vi "Dresden R2R Sputter 03.02.2018 IY24.vi"() -> ()   [LabVIEW 2009] (continued)
            n9500 = local read "Ch1_Tp_bv_do"() -> (w15535:bool)
            n9501 = local read "Ch1_Tp_bv_di"() -> (w15536:bool)
            n9502 = Exclusive Or(1:w15535, 2:w15536) -> (0:w15552:bool)
            n9503 = feedback #324() -> (w15551:bool)  [unwired: 1 in]
            n9504 = case shown="True" w15552 {
              tunnel: [TRUE FALSE] -> w15550
              tunnel: w15551 -> [_ w15589]
              tunnel: [FALSE w15586] -> w15534
              frame #0 {
              }
              frame #1 {
                n9505 = call "Elapsed Time96"("Reset"=w15589) -> ("Elapsed Time (s)"=w15588:dbl)  [unwired: 11 in, 7 out]
                n9506 = Greater?(x=w15588, y=5.0) -> (0:w15586:bool)
              }
            }
            n9507 = local write "Ch1_Tp_bv_fail"(w15534) -> ()
            n9508 = local read "Ch1_Bg_bv_di"() -> (w15533:bool)
            n9509 = local read "Ch1_Bg_bv_do"() -> (w15532:bool)
            n9510 = Exclusive Or(1:w15532, 2:w15533) -> (0:w15547:bool)
            n9511 = feedback #325() -> (w15548:bool)  [unwired: 1 in]
            n9512 = case shown="True" w15547 {
              tunnel: [TRUE FALSE] -> w15549
              tunnel: w15548 -> [_ w15582]
              tunnel: [FALSE w15579] -> w15522
              frame #0 {
              }
              frame #1 {
                n9513 = call "Elapsed Time97"("Reset"=w15582) -> ("Elapsed Time (s)"=w15581:dbl)  [unwired: 11 in, 7 out]
                n9514 = Greater?(x=w15581, y=5.0) -> (0:w15579:bool)
              }
            }
            n9515 = local write "ch1_bg_bv_fail_top"(w15522) -> ()
            n9516 = local write "Ch1_Bg_bv_fail"(w15522) -> ()
            n9517 = local read "Ch1_Ch_vbv_do"() -> (w15530:bool)
            n9518 = local read "Ch1_Ch_vbv_di"() -> (w15531:bool)
            n9519 = Exclusive Or(1:w15530, 2:w15531) -> (0:w15546:bool)
            n9520 = feedback #326() -> (w15545:bool)  [unwired: 1 in]
            n9521 = case shown="True" w15546 {
              tunnel: [TRUE FALSE] -> w15544
              tunnel: w15545 -> [_ w15575]
              tunnel: [FALSE w15572] -> w15529
              frame #0 {
              }
              frame #1 {
                n9522 = call "Elapsed Time98"("Reset"=w15575) -> ("Elapsed Time (s)"=w15574:dbl)  [unwired: 11 in, 7 out]
                n9523 = Greater?(x=w15574, y=5.0) -> (0:w15572:bool)
              }
            }
            n9524 = local write "Ch1_Ch_vbv_fail"(w15529) -> ()
            n9525 = local read "Ch1_Pl_vbv_do"() -> (w15526:bool)
            n9526 = local read "Ch1_Pl_vbv_di"() -> (w15527:bool)
            n9527 = Exclusive Or(1:w15526, 2:w15527) -> (0:w15523:bool)
            n9528 = feedback #327() -> (w15543:bool)  [unwired: 1 in]
            n9529 = case shown="True" w15523 {
              tunnel: [TRUE FALSE] -> w15542
              tunnel: w15543 -> [_ w15568]
              tunnel: [FALSE w15565] -> w15528
              frame #0 {
              }
              frame #1 {
                n9530 = call "Elapsed Time100"("Reset"=w15568) -> ("Elapsed Time (s)"=w15567:dbl)  [unwired: 11 in, 7 out]
                n9531 = Greater?(x=w15567, y=5.0) -> (0:w15565:bool)
              }
            }
            n9532 = local write "Ch1_Pl_vbv_fail"(w15528) -> ()
            n9533 = local read "Ch1_Cc_on_off_di"() -> (w15525:bool)
            n9534 = local read "Ch1_Cc_on_off_do"() -> (w15524:bool)
            n9535 = feedback #328() -> (w15540:bool)  [unwired: 1 in]
            n9536 = Exclusive Or(1:w15524, 2:w15525) -> (0:w15541:bool)
            n9537 = case shown="True" w15541 {
              tunnel: [TRUE FALSE] -> w15539
              tunnel: w15540 -> [_ w15561]
              tunnel: [FALSE w15558] -> w15521
              frame #0 {
              }
              frame #1 {
                n9538 = call "Elapsed Time102"("Reset"=w15561) -> ("Elapsed Time (s)"=w15560:dbl)  [unwired: 11 in, 7 out]
                n9539 = Greater?(x=w15560, y=5.0) -> (0:w15558:bool)
              }
            }
            n9540 = local write "ch1_cc_fail_top"(w15521) -> ()
            n9541 = local write "Ch1_Ch_cc_fail"(w15521) -> ()
          }
        }
        n9542 = case shown="False" w15450 {
          frame #0 {
            n9543 = local read "Ch1_Sov_Ar_do"() -> (w15492:bool)
            n9544 = local read "Ch1_Sov_Ar_di"() -> (w15493:bool)
            n9545 = Exclusive Or(1:w15492, 2:w15493) -> (0:w15494:bool)
            n9546 = feedback #329() -> (w15495:bool)  [unwired: 1 in]
            n9547 = case shown="True" w15494 {
              tunnel: [TRUE FALSE] -> w15496
              tunnel: w15495 -> [_ w15516]
              tunnel: [FALSE w15513] -> w15479
              frame #0 {
              }
              frame #1 {
                n9548 = call "Elapsed Time103"("Reset"=w15516) -> ("Elapsed Time (s)"=w15515:dbl)  [unwired: 11 in, 7 out]
                n9549 = Greater?(x=w15515, y=5.0) -> (0:w15513:bool)
              }
            }
            n9550 = local write "ch1_sov_Ar_fail_top"(w15479) -> ()
            n9551 = local read "Ch1_Trns_gv_open_di"() -> (w15488:bool)
            n9552 = local read "Ch1_Trns_gv_open_do"() -> (w15487:bool)
            n9553 = Exclusive Or(1:w15487, 2:w15488) -> (0:w15491:bool)
            n9554 = feedback #330() -> (w15490:bool)  [unwired: 1 in]
            n9555 = case shown="True" w15491 {
              tunnel: [TRUE FALSE] -> w15489
              tunnel: w15490 -> [_ w15509]
              tunnel: [FALSE w15506] -> w15486
              frame #0 {
              }
              frame #1 {
                n9556 = call "Elapsed Time135"("Reset"=w15509) -> ("Elapsed Time (s)"=w15508:dbl)  [unwired: 11 in, 7 out]
                n9557 = Greater?(x=w15508, y=60.0) -> (0:w15506:bool)
              }
            }
            n9558 = local write "Trns_gv1_2_fail"(w15486) -> ()
            n9559 = local write "gv top failed_ch2_1"(w15486) -> ()
            n9560 = local write "gv front failed_ch2_1"(w15486) -> ()
            n9561 = local write "gv top failed ch1"(w15486) -> ()
            n9562 = local write "gv front failed ch1_2"(w15486) -> ()
            n9563 = local read "Ch1_Cst_fix_down_di"() -> (w15484:bool)
            n9564 = local read "Ch1_Cst_fix_do"() -> (w15485:bool)
            n9565 = Exclusive Or(1:w15484, 2:w15485) -> (0:w15481:bool)
            n9566 = feedback #331() -> (w15483:bool)  [unwired: 1 in]
            n9567 = case shown="True" w15481 {
              tunnel: [TRUE FALSE] -> w15482
              tunnel: w15483 -> [_ w15502]
              tunnel: [FALSE w15499] -> w15480
              frame #0 {
              }
              frame #1 {
                n9568 = call "Elapsed Time186"("Reset"=w15502) -> ("Elapsed Time (s)"=w15501:dbl)  [unwired: 11 in, 7 out]
                n9569 = Greater?(x=w15501, y=60.0) -> (0:w15499:bool)
              }
            }
            n9570 = local write "chamber 1 top piston failed ch1"(w15480) -> ()
          }
          frame #1 {
            w15518 = TRUE
            n9571 = local write "Trns_gv1_2_fail"(w15518) -> ()
            n9572 = local write "ch1_sov_Ar_fail_top"(w15518) -> ()
            n9573 = local write "gv top failed_ch2_1"(w15518) -> ()
            n9574 = local write "gv front failed_ch2_1"(w15518) -> ()
            n9575 = local write "gv top failed ch1"(w15518) -> ()
            n9576 = local write "gv front failed ch1_2"(w15518) -> ()
            n9577 = local write "chamber 1 top piston failed ch1"(w15518) -> ()
          }
        }
        n9578 = case shown="True" w15448 {
          frame #0 {
            n9579 = disable-structure shown="Disabled" {
              frame #0 {
                n9580 = local read "Ch1_Right_limit_di"() -> (w15454:bool)
                n9581 = local read "Ch1_Do_4_4"() -> (w15455:bool)
                n9582 = Exclusive Or(1:w15455, 2:w15454) -> (0:w15453:bool)
                n9583 = feedback #332() -> (w15452:bool)  [unwired: 1 in]
                n9584 = case shown="True" w15453 {
                  tunnel: [TRUE FALSE] -> w15451
                  tunnel: w15452 -> [_ w15462]
                  tunnel: [FALSE w15459] -> w15456
                  frame #0 {
                  }
                  frame #1 {
                    n9585 = call "Elapsed Time108"("Reset"=w15462) -> ("Elapsed Time (s)"=w15461:dbl)  [unwired: 11 in, 7 out]
                    n9586 = Greater?(x=w15461, y=5.0) -> (0:w15459:bool)
                  }
                }
                n9587 = local write "Ch1_Bp_bv_fail_R"(w15456) -> ()
              }
              frame #1 {
              }
            }
          }
          frame #1 {
            n9588 = disable-structure shown="Disabled" {
              frame #0 {
                n9589 = local write "Ch1_Bp_bv_fail_R"(FALSE ("Bp_bv_fail(ch1)R")) -> ()
              }
              frame #1 {
              }
            }
          }
        }
      }
    }
    n9590 = Wait Until Next ms Multiple(millisecond multiple=u32 200) -> ()  [unwired: 1 out]
  }
  n9591 = while {
    tunnel: w804 -> [w15654]
    tunnel: w803 -> [w15653]
    tunnel: [w15652] -> w802
    tunnel: [w15651] -> w801
    tunnel: w737 -> [w15606]
    tunnel: w736 -> [w15605]
    tunnel: [w15604] -> w735
    tunnel: [w15603] -> w734
    tunnel: w27 -> [w15602]
    tunnel: w26 -> [w15601]
    tunnel: [w15599] -> w25
    tunnel: [w15598] -> w24
    stop <- i16? 0 stop-if-true
    # "According to manual, all starting addresses must be used increment"
    n9592 = Wait Until Next ms Multiple(millisecond multiple=i32? 300) -> ()  [unwired: 1 out]
    n9593 = Or(x="TC1_set", y="TC1_auto_set") -> (x .or. y?=w15636)
    n9594 = Or(x="TC2_set", y="TC2_auto_set") -> (x .or. y?=w15612)
    n9595 = Build Array(i16? 0, w15636, "TC1_open_loop_set", "TC1_close_loop_set", "TC1_P_set", "TC1_I_set", "TC1_D_set", "TC1_speed_gain_set", "TC1_speed_coefficient_set", "TC1_overspeed_set", "TC1_AO1_upper_limit_set", "TC1_AO1_bottom_limit_set", "TC1_AO1_polarity(neg_to_pos)", "TC1_AO1_polarity(pos_to_neg)", "TC1_display_tension_set", "TC1_display_AO1_set", "TC1_display_tension_actual", "TC1_display_AO1_actual", "TC1_tare_function") -> (w15657)
    n9596 = Build Array(i16? 0, w15612, "TC2_open_loop_set", "TC2_close_loop_set", "TC2_P_set", "TC2_I_set", "TC2_D_set", "TC2_speed_gain_set", "TC2_speed_coefficient_set", "TC2_overspeed_set", "TC2_AO1_upper_limit_set", "TC2_AO1_bottom_limit_set", "TC2_AO1_polarity(neg_to_pos)", "TC2_AO1_polarity(pos_to_neg)", "TC2_display_tension_set", "TC2_display_AO1_set", "TC2_display_tension_actual", "TC2_display_AO1_actual", "TC2_tare_function") -> (w15629)
    n9597 = Boolean Array To Number(Boolean array=w15657) -> (number=w15658)
    n9598 = Boolean Array To Number(Boolean array=w15629) -> (number=w15630)
    n9599 = case shown="True" "Counter_reset" {
      tunnel: w15602 -> [w15667 w15676]
      tunnel: w15601 -> [w15666 w15675]
      tunnel: [w15665 w15674] -> w15599
      tunnel: [w15664 w15673] -> w15598
      frame #0 {
        n9600 = call-poly <vilib>:"MB Serial Master Query (poly).vi"(0:w15667, 1:i16? 1000 ("Starting Address"), 2:i16? 13 ("Quantity"), 5:w15666, 6:data[3B] ("Serial Parameters")) -> (14:w15665, 15:w15663, 19:w15664)  [unwired: 1 in, 11 out]
        n9601 = Index Array(array=w15663, index=i32? 3) -> (element=→"Counter_read_data")
      }
      frame #1 {
        n9602 = local write "Counter_reset"(i16? 0 ("Counter_reset")) -> ()
        n9603 = call-poly <vilib>:"MB Serial Master Query (poly).vi"(0:w15676, 1:data[3B] ("Starting Address"), 2:T/1, 5:w15675, 6:data[3B] ("Serial Parameters")) -> (14:w15674, 19:w15673)  [unwired: 1 in, 12 out]
      }
    }
    n9604 = Mantissa & Exponent(0:w15658) -> (2:w15656)  [unwired: 1 out]
    n9605 = Mantissa & Exponent(0:w15630) -> (2:w15628)  [unwired: 1 out]
    n9606 = case shown="1" w15656 {
      tunnel: w15654 -> [w16130 w16153 w16175 w16197 w16219 w16241 w16263 w16285 w16307 w16329 w16351 w16373 w16395 w16417 w16439 w16461 w16483 w16505 w16527]
      tunnel: w15653 -> [w16129 w16152 w16174 w16196 w16218 w16240 w16262 w16284 w16306 w16328 w16350 w16372 w16394 w16416 w16438 w16460 w16482 w16504 w16526]
      tunnel: [w16128 w16156 w16178 w16200 w16222 w16244 w16266 w16288 w16310 w16332 w16354 w16376 w16398 w16420 w16442 w16464 w16486 w16508 w16529] -> w15652
      tunnel: [w16106 w16155 w16177 w16199 w16221 w16243 w16265 w16287 w16309 w16331 w16353 w16375 w16397 w16419 w16441 w16463 w16485 w16507 w16528] -> w15651
      frame #0 {
        n9607 = Increment(x=i16? 296 ("Starting Address")) -> (x+1=w16126)
        n9608 = call <vilib>:"MB Serial Master Query Read Holding Registers (poly).vi"(0:w16130, 1:w16126, 2:i16? 4 ("Quantity"), 5:w16129, 6:data[3B] ("Serial Parameters")) -> (14:w16128, 15:w16107, 19:w16106)  [unwired: 11 in, 1 out]
        n9609 = Index Array(array=w16107, index=data[5B]) -> (element=w16123)
        n9610 = Index Array(array=w16107, index=i32? 2) -> (element=w16121)
        n9611 = Index Array(array=w16107, index=i32? 6) -> (element=w16113)
        n9612 = Type Cast(type=data[5B], x=w16123) -> (*(type *) &x=w16105)
        "TC1_reading_set_value" <- w16105
        n9613 = Type Cast(type=data[5B], x=w16121) -> (*(type *) &x=w16115)
        n9614 = Type Cast(type=data[5B], x=w16113) -> (*(type *) &x=w16109)
        n9615 = Greater?(x=w16115, y=sgl? 0.1) -> (0:w16117)
        n9616 = Divide(x=w16109, y=sgl? 10) -> (x/y=→"TC1_reading_ao_value")
        n9617 = Select(t=w16115, s=w16117, f=data[5B]) -> (s? t:f=→"TC1_measure_value")
        n9618 = stacked-sequence {
          tunnel: w16105 -> [w16132]
          frame #0 {
            n9619 = feedback #333() -> (w16144)  [unwired: 1 in]
            n9620 = feedback #334() -> (w16142)  [unwired: 1 in]
            n9621 = feedback #335() -> (w16141)  [unwired: 1 in]
            n9622 = feedback #336() -> (w16140)  [unwired: 1 in]
            n9623 = feedback #337() -> (w16139)  [unwired: 1 in]
            n9624 = feedback #338() -> (w16138)  [unwired: 1 in]
            n9625 = feedback #339() -> (w16137)  [unwired: 1 in]
            n9626 = feedback #340() -> (w16135)  [unwired: 1 in]
            n9627 = feedback #341() -> (w16136)  [unwired: 1 in]
            n9628 = Compound Arithmetic op=ADD(w16132, w16144, w16142, w16141, w16140, w16139, w16138, w16137, w16135, w16136) -> (w16143)
            n9629 = Divide(x=w16143, y=dbl? 10.0) -> (x/y=→"TC1_Tension_read_set")
          }
        }
      }
      frame #1 {
        w16145 = i16? 0 ("TC1_set")
        w16154 = data[3B] ("Serial Parameters")
        n9630 = Type Cast(type=data[3B], x="TC1_set_value") -> (*(type *) &x=w16146)
        n9631 = Build Array(w16146) -> (w16147)
        n9632 = Increment(x=i16? 142) -> (x+1=w16151)
        n9633 = call <vilib>:"MB Serial Master Query Write Multiple Registers (poly).vi"(0:w16153, 1:w16151, 2:w16147, 5:w16152, 6:w16154) -> (14:w16161, 19:w16160)  [unwired: 12 in, 1 out]
        n9634 = local write "TC1_auto_set"(w16145) -> ()
        n9635 = local write "TC1_set"(w16145) -> ()
        n9636 = Build Array(i32? 49152 ("element")) -> (w16159)
        n9637 = call <vilib>:"MB Serial Master Query Write Multiple Registers (poly).vi"(0:w16161, 1:i16? 320 ("Starting Address"), 2:w16159, 5:w16160, 6:w16154) -> (14:w16165, 19:w16166)  [unwired: 12 in, 1 out]
        n9638 = Build Array(i32? 49407 ("element")) -> (w16162)
        n9639 = call <vilib>:"MB Serial Master Query Write Multiple Registers (poly).vi"(0:w16165, 1:i16? 320 ("Starting Address"), 2:w16162, 5:w16166, 6:w16154) -> (14:w16156, 19:w16155)  [unwired: 12 in, 1 out]
      }
      frame #2 {
        w16176 = data[3B] ("Serial Parameters")
        n9640 = Type Cast(type=data[3B], x="TC1_open_loop_coefficient") -> (*(type *) &x=w16168)
        n9641 = Build Array(w16168) -> (w16169)
        n9642 = Increment(x=i16? 82) -> (x+1=w16173)
        n9643 = call <vilib>:"MB Serial Master Query Write Multiple Registers (poly).vi"(0:w16175, 1:w16173, 2:w16169, 5:w16174, 6:w16176) -> (14:w16183, 19:w16182)  [unwired: 12 in, 1 out]
        n9644 = local write "TC1_open_loop_set"(i16? 0 ("TC1_open_loop_set")) -> ()
        n9645 = Build Array(i32? 49152 ("element")) -> (w16181)
        n9646 = call <vilib>:"MB Serial Master Query Write Multiple Registers (poly).vi"(0:w16183, 1:i16? 320 ("Starting Address"), 2:w16181, 5:w16182, 6:w16176) -> (14:w16187, 19:w16188)  [unwired: 12 in, 1 out]
        n9647 = Build Array(i32? 49407 ("element")) -> (w16184)
        n9648 = call <vilib>:"MB Serial Master Query Write Multiple Registers (poly).vi"(0:w16187, 1:i16? 320 ("Starting Address"), 2:w16184, 5:w16188, 6:w16176) -> (14:w16178, 19:w16177)  [unwired: 12 in, 1 out]
      }
      frame #3 {
        w16198 = data[3B] ("Serial Parameters")
        n9649 = Type Cast(type=data[3B], x="TC1_close_loop_coefficient") -> (*(type *) &x=w16190)
        n9650 = Build Array(w16190) -> (w16191)
        n9651 = Increment(x=i16? 84) -> (x+1=w16195)
        n9652 = call <vilib>:"MB Serial Master Query Write Multiple Registers (poly).vi"(0:w16197, 1:w16195, 2:w16191, 5:w16196, 6:w16198) -> (14:w16205, 19:w16204)  [unwired: 12 in, 1 out]
        n9653 = local write "TC1_close_loop_set"(i16? 0 ("TC1_close_loop_set")) -> ()
        n9654 = Build Array(i32? 49152 ("element")) -> (w16203)
        n9655 = call <vilib>:"MB Serial Master Query Write Multiple Registers (poly).vi"(0:w16205, 1:i16? 320 ("Starting Address"), 2:w16203, 5:w16204, 6:w16198) -> (14:w16209, 19:w16210)  [unwired: 12 in, 1 out]
        n9656 = Build Array(i32? 49407 ("element")) -> (w16206)
        n9657 = call <vilib>:"MB Serial Master Query Write Multiple Registers (poly).vi"(0:w16209, 1:i16? 320 ("Starting Address"), 2:w16206, 5:w16210, 6:w16198) -> (14:w16200, 19:w16199)  [unwired: 12 in, 1 out]
      }
      frame #4 {
        w16220 = data[3B] ("Serial Parameters")
        n9658 = Type Cast(type=data[3B], x="TC1_P_coefficient") -> (*(type *) &x=w16212)
        n9659 = Build Array(w16212) -> (w16213)
        n9660 = Increment(x=i16? 108) -> (x+1=w16217)
        n9661 = call <vilib>:"MB Serial Master Query Write Multiple Registers (poly).vi"(0:w16219, 1:w16217, 2:w16213, 5:w16218, 6:w16220) -> (14:w16227, 19:w16226)  [unwired: 12 in, 1 out]
        n9662 = local write "TC1_P_set"(i16? 0 ("TC1_P_set")) -> ()
        n9663 = Build Array(i32? 49152 ("element")) -> (w16225)
        n9664 = call <vilib>:"MB Serial Master Query Write Multiple Registers (poly).vi"(0:w16227, 1:i16? 320 ("Starting Address"), 2:w16225, 5:w16226, 6:w16220) -> (14:w16231, 19:w16232)  [unwired: 12 in, 1 out]
        n9665 = Build Array(i32? 49407 ("element")) -> (w16228)
        n9666 = call <vilib>:"MB Serial Master Query Write Multiple Registers (poly).vi"(0:w16231, 1:i16? 320 ("Starting Address"), 2:w16228, 5:w16232, 6:w16220) -> (14:w16222, 19:w16221)  [unwired: 12 in, 1 out]
      }
      frame #5 {
        w16242 = data[3B] ("Serial Parameters")
        n9667 = Type Cast(type=data[3B], x="TC1_I_coefficient") -> (*(type *) &x=w16234)
        n9668 = Build Array(w16234) -> (w16235)
        n9669 = Increment(x=i16? 110) -> (x+1=w16239)
        n9670 = call <vilib>:"MB Serial Master Query Write Multiple Registers (poly).vi"(0:w16241, 1:w16239, 2:w16235, 5:w16240, 6:w16242) -> (14:w16249, 19:w16248)  [unwired: 12 in, 1 out]
        n9671 = local write "TC1_I_set"(i16? 0 ("TC1_I_set")) -> ()
        n9672 = Build Array(i32? 49152 ("element")) -> (w16247)
        n9673 = call <vilib>:"MB Serial Master Query Write Multiple Registers (poly).vi"(0:w16249, 1:i16? 320 ("Starting Address"), 2:w16247, 5:w16248, 6:w16242) -> (14:w16253, 19:w16254)  [unwired: 12 in, 1 out]
        n9674 = Build Array(i32? 49407 ("element")) -> (w16250)
        n9675 = call <vilib>:"MB Serial Master Query Write Multiple Registers (poly).vi"(0:w16253, 1:i16? 320 ("Starting Address"), 2:w16250, 5:w16254, 6:w16242) -> (14:w16244, 19:w16243)  [unwired: 12 in, 1 out]
      }
      frame #6 {
        w16264 = data[3B] ("Serial Parameters")
        n9676 = Type Cast(type=data[3B], x="TC1_D_coefficient") -> (*(type *) &x=w16256)
        n9677 = Build Array(w16256) -> (w16257)
        n9678 = Increment(x=i16? 112) -> (x+1=w16261)
        n9679 = call <vilib>:"MB Serial Master Query Write Multiple Registers (poly).vi"(0:w16263, 1:w16261, 2:w16257, 5:w16262, 6:w16264) -> (14:w16271, 19:w16270)  [unwired: 12 in, 1 out]
        n9680 = local write "TC1_D_set"(i16? 0 ("TC1_D_set")) -> ()
        n9681 = Build Array(i32? 49152 ("element")) -> (w16269)
        n9682 = call <vilib>:"MB Serial Master Query Write Multiple Registers (poly).vi"(0:w16271, 1:i16? 320 ("Starting Address"), 2:w16269, 5:w16270, 6:w16264) -> (14:w16275, 19:w16276)  [unwired: 12 in, 1 out]
        n9683 = Build Array(i32? 49407 ("element")) -> (w16272)
        n9684 = call <vilib>:"MB Serial Master Query Write Multiple Registers (poly).vi"(0:w16275, 1:i16? 320 ("Starting Address"), 2:w16272, 5:w16276, 6:w16264) -> (14:w16266, 19:w16265)  [unwired: 12 in, 1 out]
      }
      frame #7 {
        w16286 = data[3B] ("Serial Parameters")
        n9685 = Type Cast(type=data[3B], x="TC1_speed_gain_value") -> (*(type *) &x=w16278)
        n9686 = Build Array(w16278) -> (w16279)
        n9687 = Increment(x=i16? 126) -> (x+1=w16283)
        n9688 = call <vilib>:"MB Serial Master Query Write Multiple Registers (poly).vi"(0:w16285, 1:w16283, 2:w16279, 5:w16284, 6:w16286) -> (14:w16293, 19:w16292)  [unwired: 12 in, 1 out]
        n9689 = local write "TC1_speed_gain_set"(i16? 0 ("TC1_speed_gain_set")) -> ()
        n9690 = Build Array(i32? 49152 ("element")) -> (w16291)
        n9691 = call <vilib>:"MB Serial Master Query Write Multiple Registers (poly).vi"(0:w16293, 1:i16? 320 ("Starting Address"), 2:w16291, 5:w16292, 6:w16286) -> (14:w16297, 19:w16298)  [unwired: 12 in, 1 out]
        n9692 = Build Array(i32? 49407 ("element")) -> (w16294)
        n9693 = call <vilib>:"MB Serial Master Query Write Multiple Registers (poly).vi"(0:w16297, 1:i16? 320 ("Starting Address"), 2:w16294, 5:w16298, 6:w16286) -> (14:w16288, 19:w16287)  [unwired: 12 in, 1 out]
      }
      frame #8 {
        w16308 = data[3B] ("Serial Parameters")
        n9694 = Type Cast(type=data[3B], x="TC1_speed_coefficient_value") -> (*(type *) &x=w16300)
        n9695 = Build Array(w16300) -> (w16301)
        n9696 = Increment(x=i16? 128) -> (x+1=w16305)
        n9697 = call <vilib>:"MB Serial Master Query Write Multiple Registers (poly).vi"(0:w16307, 1:w16305, 2:w16301, 5:w16306, 6:w16308) -> (14:w16315, 19:w16314)  [unwired: 12 in, 1 out]
        n9698 = local write "TC1_speed_coefficient_set"(i16? 0 ("TC1_speed_coefficient_set")) -> ()
        n9699 = Build Array(i32? 49152 ("element")) -> (w16313)
        n9700 = call <vilib>:"MB Serial Master Query Write Multiple Registers (poly).vi"(0:w16315, 1:i16? 320 ("Starting Address"), 2:w16313, 5:w16314, 6:w16308) -> (14:w16319, 19:w16320)  [unwired: 12 in, 1 out]
        n9701 = Build Array(i32? 49407 ("element")) -> (w16316)
        n9702 = call <vilib>:"MB Serial Master Query Write Multiple Registers (poly).vi"(0:w16319, 1:i16? 320 ("Starting Address"), 2:w16316, 5:w16320, 6:w16308) -> (14:w16310, 19:w16309)  [unwired: 12 in, 1 out]
      }
      frame #9 {
        w16330 = data[3B] ("Serial Parameters")
        n9703 = Type Cast(type=data[3B], x="TC1_overspeed_value") -> (*(type *) &x=w16322)
        n9704 = Build Array(w16322) -> (w16323)
        n9705 = Increment(x=i16? 130) -> (x+1=w16327)
        n9706 = call <vilib>:"MB Serial Master Query Write Multiple Registers (poly).vi"(0:w16329, 1:w16327, 2:w16323, 5:w16328, 6:w16330) -> (14:w16337, 19:w16336)  [unwired: 12 in, 1 out]
        n9707 = local write "TC1_overspeed_set"(i16? 0 ("TC1_overspeed_set")) -> ()
        n9708 = Build Array(i32? 49152 ("element")) -> (w16335)
        n9709 = call <vilib>:"MB Serial Master Query Write Multiple Registers (poly).vi"(0:w16337, 1:i16? 320 ("Starting Address"), 2:w16335, 5:w16336, 6:w16330) -> (14:w16341, 19:w16342)  [unwired: 12 in, 1 out]
        n9710 = Build Array(i32? 49407 ("element")) -> (w16338)
        n9711 = call <vilib>:"MB Serial Master Query Write Multiple Registers (poly).vi"(0:w16341, 1:i16? 320 ("Starting Address"), 2:w16338, 5:w16342, 6:w16330) -> (14:w16332, 19:w16331)  [unwired: 12 in, 1 out]
      }
      frame #10 {
        w16352 = data[3B] ("Serial Parameters")
        n9712 = Type Cast(type=data[3B], x="TC1_AO1_upper_limit_value") -> (*(type *) &x=w16344)
        n9713 = Build Array(w16344) -> (w16345)
        n9714 = Increment(x=i16? 168) -> (x+1=w16349)
        n9715 = call <vilib>:"MB Serial Master Query Write Multiple Registers (poly).vi"(0:w16351, 1:w16349, 2:w16345, 5:w16350, 6:w16352) -> (14:w16359, 19:w16358)  [unwired: 12 in, 1 out]
        n9716 = local write "TC1_AO1_upper_limit_set"(i16? 0 ("TC1_AO1_upper_limit_set")) -> ()
        n9717 = Build Array(i32? 49152 ("element")) -> (w16357)
        n9718 = call <vilib>:"MB Serial Master Query Write Multiple Registers (poly).vi"(0:w16359, 1:i16? 320 ("Starting Address"), 2:w16357, 5:w16358, 6:w16352) -> (14:w16363, 19:w16364)  [unwired: 12 in, 1 out]
        n9719 = Build Array(i32? 49407 ("element")) -> (w16360)
        n9720 = call <vilib>:"MB Serial Master Query Write Multiple Registers (poly).vi"(0:w16363, 1:i16? 320 ("Starting Address"), 2:w16360, 5:w16364, 6:w16352) -> (14:w16354, 19:w16353)  [unwired: 12 in, 1 out]
      }
      frame #11 {
        w16374 = data[3B] ("Serial Parameters")
        n9721 = Type Cast(type=data[3B], x="TC1_AO1_bottom_limit_value") -> (*(type *) &x=w16366)
        n9722 = Build Array(w16366) -> (w16367)
        n9723 = Increment(x=i16? 166) -> (x+1=w16371)
        n9724 = call <vilib>:"MB Serial Master Query Write Multiple Registers (poly).vi"(0:w16373, 1:w16371, 2:w16367, 5:w16372, 6:w16374) -> (14:w16381, 19:w16380)  [unwired: 12 in, 1 out]
        n9725 = local write "TC1_AO1_bottom_limit_set"(i16? 0 ("TC1_AO1_bottom_limit_set")) -> ()
        n9726 = Build Array(i32? 49152 ("element")) -> (w16379)
        n9727 = call <vilib>:"MB Serial Master Query Write Multiple Registers (poly).vi"(0:w16381, 1:i16? 320 ("Starting Address"), 2:w16379, 5:w16380, 6:w16374) -> (14:w16385, 19:w16386)  [unwired: 12 in, 1 out]
        n9728 = Build Array(i32? 49407 ("element")) -> (w16382)
        n9729 = call <vilib>:"MB Serial Master Query Write Multiple Registers (poly).vi"(0:w16385, 1:i16? 320 ("Starting Address"), 2:w16382, 5:w16386, 6:w16374) -> (14:w16376, 19:w16375)  [unwired: 12 in, 1 out]
      }
      frame #12 {
        w16396 = data[3B] ("Serial Parameters")
        n9730 = Type Cast(type=data[3B], x=data[5B] ("TC1_AO1_bottom_limit_value 2")) -> (*(type *) &x=w16388)
        n9731 = Build Array(w16388) -> (w16389)
        n9732 = Increment(x=i16? 198) -> (x+1=w16393)
        n9733 = call <vilib>:"MB Serial Master Query Write Multiple Registers (poly).vi"(0:w16395, 1:w16393, 2:w16389, 5:w16394, 6:w16396) -> (14:w16403, 19:w16402)  [unwired: 12 in, 1 out]
        n9734 = local write "TC1_AO1_polarity(neg_to_pos)"(i16? 0 ("TC1_AO1_polarity(neg_to_pos)")) -> ()
        n9735 = Build Array(i32? 49152 ("element")) -> (w16401)
        n9736 = call <vilib>:"MB Serial Master Query Write Multiple Registers (poly).vi"(0:w16403, 1:i16? 320 ("Starting Address"), 2:w16401, 5:w16402, 6:w16396) -> (14:w16407, 19:w16408)  [unwired: 12 in, 1 out]
        n9737 = Build Array(i32? 49407 ("element")) -> (w16404)
        n9738 = call <vilib>:"MB Serial Master Query Write Multiple Registers (poly).vi"(0:w16407, 1:i16? 320 ("Starting Address"), 2:w16404, 5:w16408, 6:w16396) -> (14:w16398, 19:w16397)  [unwired: 12 in, 1 out]
      }
      frame #13 {
        w16418 = data[3B] ("Serial Parameters")
        n9739 = Type Cast(type=data[3B], x=sgl? 1 ("TC1_AO1_bottom_limit_value 2")) -> (*(type *) &x=w16410)
        n9740 = Build Array(w16410) -> (w16411)
        n9741 = Increment(x=i16? 198) -> (x+1=w16415)
        n9742 = call <vilib>:"MB Serial Master Query Write Multiple Registers (poly).vi"(0:w16417, 1:w16415, 2:w16411, 5:w16416, 6:w16418) -> (14:w16425, 19:w16424)  [unwired: 12 in, 1 out]
        n9743 = local write "TC1_AO1_polarity(pos_to_neg)"(i16? 0 ("TC1_AO1_polarity(pos_to_neg)")) -> ()
        n9744 = Build Array(i32? 49152 ("element")) -> (w16423)
        n9745 = call <vilib>:"MB Serial Master Query Write Multiple Registers (poly).vi"(0:w16425, 1:i16? 320 ("Starting Address"), 2:w16423, 5:w16424, 6:w16418) -> (14:w16429, 19:w16430)  [unwired: 12 in, 1 out]
        n9746 = Build Array(i32? 49407 ("element")) -> (w16426)
        n9747 = call <vilib>:"MB Serial Master Query Write Multiple Registers (poly).vi"(0:w16429, 1:i16? 320 ("Starting Address"), 2:w16426, 5:w16430, 6:w16418) -> (14:w16420, 19:w16419)  [unwired: 12 in, 1 out]
      }
      frame #14 {
        w16440 = data[3B] ("Serial Parameters")
        n9748 = Type Cast(type=data[3B], x=sgl? 2 ("TC1_AO1_bottom_limit_value 2")) -> (*(type *) &x=w16432)
        n9749 = Build Array(w16432) -> (w16433)
        n9750 = Increment(x=i16? 8) -> (x+1=w16437)
        n9751 = call <vilib>:"MB Serial Master Query Write Multiple Registers (poly).vi"(0:w16439, 1:w16437, 2:w16433, 5:w16438, 6:w16440) -> (14:w16447, 19:w16446)  [unwired: 12 in, 1 out]
        n9752 = local write "TC1_display_tension_set"(i16? 0 ("TC1_display_tension")) -> ()
        n9753 = Build Array(i32? 49152 ("element")) -> (w16445)
        n9754 = call <vilib>:"MB Serial Master Query Write Multiple Registers (poly).vi"(0:w16447, 1:i16? 320 ("Starting Address"), 2:w16445, 5:w16446, 6:w16440) -> (14:w16451, 19:w16452)  [unwired: 12 in, 1 out]
        n9755 = Build Array(i32? 49407 ("element")) -> (w16448)
        n9756 = call <vilib>:"MB Serial Master Query Write Multiple Registers (poly).vi"(0:w16451, 1:i16? 320 ("Starting Address"), 2:w16448, 5:w16452, 6:w16440) -> (14:w16442, 19:w16441)  [unwired: 12 in, 1 out]
      }
      frame #15 {
        w16462 = data[3B] ("Serial Parameters")
        n9757 = Type Cast(type=data[3B], x=sgl? 5 ("TC1_AO1_bottom_limit_value 2")) -> (*(type *) &x=w16454)
        n9758 = Build Array(w16454) -> (w16455)
        n9759 = Increment(x=i16? 8) -> (x+1=w16459)
        n9760 = call <vilib>:"MB Serial Master Query Write Multiple Registers (poly).vi"(0:w16461, 1:w16459, 2:w16455, 5:w16460, 6:w16462) -> (14:w16469, 19:w16468)  [unwired: 12 in, 1 out]
        n9761 = local write "TC1_display_AO1_set"(i16? 0 ("TC1_display_AO1")) -> ()
        n9762 = Build Array(i32? 49152 ("element")) -> (w16467)
        n9763 = call <vilib>:"MB Serial Master Query Write Multiple Registers (poly).vi"(0:w16469, 1:i16? 320 ("Starting Address"), 2:w16467, 5:w16468, 6:w16462) -> (14:w16473, 19:w16474)  [unwired: 12 in, 1 out]
        n9764 = Build Array(i32? 49407 ("element")) -> (w16470)
        n9765 = call <vilib>:"MB Serial Master Query Write Multiple Registers (poly).vi"(0:w16473, 1:i16? 320 ("Starting Address"), 2:w16470, 5:w16474, 6:w16462) -> (14:w16464, 19:w16463)  [unwired: 12 in, 1 out]
      }
      frame #16 {
        w16484 = data[3B] ("Serial Parameters")
        n9766 = Type Cast(type=data[3B], x=sgl? 4 ("TC1_AO1_bottom_limit_value 2")) -> (*(type *) &x=w16476)
        n9767 = Build Array(w16476) -> (w16477)
        n9768 = Increment(x=i16? 10) -> (x+1=w16481)
        n9769 = call <vilib>:"MB Serial Master Query Write Multiple Registers (poly).vi"(0:w16483, 1:w16481, 2:w16477, 5:w16482, 6:w16484) -> (14:w16491, 19:w16490)  [unwired: 12 in, 1 out]
        n9770 = local write "TC1_display_tension_actual"(i16? 0 ("TC1_display_tension")) -> ()
        n9771 = Build Array(i32? 49152 ("element")) -> (w16489)
        n9772 = call <vilib>:"MB Serial Master Query Write Multiple Registers (poly).vi"(0:w16491, 1:i16? 320 ("Starting Address"), 2:w16489, 5:w16490, 6:w16484) -> (14:w16495, 19:w16496)  [unwired: 12 in, 1 out]
        n9773 = Build Array(i32? 49407 ("element")) -> (w16492)
        n9774 = call <vilib>:"MB Serial Master Query Write Multiple Registers (poly).vi"(0:w16495, 1:i16? 320 ("Starting Address"), 2:w16492, 5:w16496, 6:w16484) -> (14:w16486, 19:w16485)  [unwired: 12 in, 1 out]
      }
      frame #17 {
        w16506 = data[3B] ("Serial Parameters")
        n9775 = Type Cast(type=data[3B], x=data[5B] ("TC1_AO1_bottom_limit_value 2")) -> (*(type *) &x=w16498)
        n9776 = Build Array(w16498) -> (w16499)
        n9777 = Increment(x=i16? 10) -> (x+1=w16503)
        n9778 = call <vilib>:"MB Serial Master Query Write Multiple Registers (poly).vi"(0:w16505, 1:w16503, 2:w16499, 5:w16504, 6:w16506) -> (14:w16513, 19:w16512)  [unwired: 12 in, 1 out]
        n9779 = local write "TC1_display_AO1_actual"(i16? 0 ("TC1_display_tension")) -> ()
        n9780 = Build Array(i32? 49152 ("element")) -> (w16511)
        n9781 = call <vilib>:"MB Serial Master Query Write Multiple Registers (poly).vi"(0:w16513, 1:i16? 320 ("Starting Address"), 2:w16511, 5:w16512, 6:w16506) -> (14:w16517, 19:w16518)  [unwired: 12 in, 1 out]
        n9782 = Build Array(i32? 49407 ("element")) -> (w16514)
        n9783 = call <vilib>:"MB Serial Master Query Write Multiple Registers (poly).vi"(0:w16517, 1:i16? 320 ("Starting Address"), 2:w16514, 5:w16518, 6:w16506) -> (14:w16508, 19:w16507)  [unwired: 12 in, 1 out]
      }
      frame #18 {
        n9784 = Build Array(i16? 21767 ("Starting Address")) -> (w16521)
        n9785 = call <vilib>:"MB Serial Master Query Write Multiple Registers (poly).vi"(0:w16527, 1:i16? 322 ("Starting Address"), 2:w16521, 5:w16526, 6:data[3B] ("Serial Parameters")) -> (14:w16523, 19:w16522)  [unwired: 12 in, 1 out]
        n9786 = local write "TC1_tare_function"(i16? 0 ("TC1_tare_function")) -> ()
        n9787 = Build Array(i32? 49407 ("element")) -> (w16530)
        n9788 = call <vilib>:"MB Serial Master Query Write Multiple Registers (poly).vi"(0:w16523, 1:i16? 320 ("Starting Address"), 2:w16530, 5:w16522) -> (14:w16529, 19:w16528)  [unwired: 13 in, 1 out]
      }
    }
    n9789 = case shown="1" w15628 {
      tunnel: w15606 -> [w15702 w15725 w15747 w15769 w15791 w15813 w15835 w15857 w15879 w15901 w15923 w15945 w15967 w15989 w16011 w16033 w16055 w16077 w16099]
      tunnel: w15605 -> [w15701 w15724 w15746 w15768 w15790 w15812 w15834 w15850 w15878 w15900 w15922 w15944 w15966 w15988 w16010 w16032 w16054 w16076 w16098]
      tunnel: [w15700 w15728 w15750 w15772 w15794 w15816 w15838 w15860 w15882 w15904 w15926 w15948 w15970 w15992 w16014 w16036 w16058 w16080 w16101] -> w15604
      tunnel: [w15689 w15727 w15749 w15771 w15793 w15815 w15837 w15859 w15881 w15903 w15925 w15947 w15969 w15991 w16013 w16035 w16057 w16079 w16100] -> w15603
      frame #0 {
        n9790 = Increment(x=i16? 296 ("Starting Address")) -> (x+1=w15698)
        n9791 = call <vilib>:"MB Serial Master Query Read Holding Registers (poly).vi"(0:w15702, 1:w15698, 2:i16? 4 ("Quantity"), 5:w15701, 6:data[3B] ("Serial Parameters")) -> (14:w15700, 15:w15681, 19:w15689)  [unwired: 11 in, 1 out]
        n9792 = Index Array(array=w15681, index=data[5B]) -> (element=w15695)
        n9793 = Index Array(array=w15681, index=i32? 8) -> (element=w15682)
        n9794 = Index Array(array=w15681, index=i32? 2) -> (element=w15693)
        n9795 = Type Cast(type=data[5B], x=w15695) -> (*(type *) &x=w15679)
        "TC2_reading_set_value" <- w15679
        n9796 = Type Cast(type=data[5B], x=w15682) -> (*(type *) &x=→"TC1_reading_ao_value 2")
        n9797 = Type Cast(type=data[5B], x=w15693) -> (*(type *) &x=w15686)
        n9798 = Greater?(x=w15686, y=sgl? 0.1) -> (0:w15688)
        n9799 = Select(t=w15686, s=w15688, f=data[5B]) -> (s? t:f=→"TC2_measure_value")
        n9800 = stacked-sequence {
          tunnel: w15679 -> [w15704]
          frame #0 {
            n9801 = feedback #342() -> (w15706)  [unwired: 1 in]
            n9802 = feedback #343() -> (w15707)  [unwired: 1 in]
            n9803 = feedback #344() -> (w15708)  [unwired: 1 in]
            n9804 = feedback #345() -> (w15709)  [unwired: 1 in]
            n9805 = feedback #346() -> (w15710)  [unwired: 1 in]
            n9806 = feedback #347() -> (w15711)  [unwired: 1 in]
            n9807 = feedback #348() -> (w15712)  [unwired: 1 in]
            n9808 = feedback #349() -> (w15714)  [unwired: 1 in]
            n9809 = feedback #350() -> (w15713)  [unwired: 1 in]
            n9810 = Compound Arithmetic op=ADD(w15704, w15706, w15707, w15708, w15709, w15710, w15711, w15712, w15714, w15713) -> (w15705)
            n9811 = Divide(x=w15705, y=dbl? 10.0) -> (x/y=→"TC2_Tension_read_set")
          }
        }
      }
      frame #1 {
        w15717 = i16? 0 ("TC2_set")
        w15726 = data[3B] ("Serial Parameters")
        n9812 = Type Cast(type=data[3B], x="TC2_set_value") -> (*(type *) &x=w15718)
        n9813 = Build Array(w15718) -> (w15719)
        n9814 = Increment(x=i16? 142) -> (x+1=w15723)
        n9815 = call <vilib>:"MB Serial Master Query Write Multiple Registers (poly).vi"(0:w15725, 1:w15723, 2:w15719, 5:w15724, 6:w15726) -> (14:w15733, 19:w15732)  [unwired: 12 in, 1 out]
        n9816 = local write "TC2_auto_set"(w15717) -> ()
        n9817 = local write "TC2_set"(w15717) -> ()
        n9818 = Build Array(i32? 49152 ("element")) -> (w15731)
        n9819 = call <vilib>:"MB Serial Master Query Write Multiple Registers (poly).vi"(0:w15733, 1:i16? 320 ("Starting Address"), 2:w15731, 5:w15732, 6:w15726) -> (14:w15737, 19:w15738)  [unwired: 12 in, 1 out]
        n9820 = Build Array(i32? 49407 ("element")) -> (w15734)
        n9821 = call <vilib>:"MB Serial Master Query Write Multiple Registers (poly).vi"(0:w15737, 1:i16? 320 ("Starting Address"), 2:w15734, 5:w15738, 6:w15726) -> (14:w15728, 19:w15727)  [unwired: 12 in, 1 out]
      }
      frame #2 {
        w15748 = data[3B] ("Serial Parameters")
        n9822 = Type Cast(type=data[3B], x="TC2_open_loop_coefficient") -> (*(type *) &x=w15740)
        n9823 = Build Array(w15740) -> (w15741)
        n9824 = Increment(x=i16? 82) -> (x+1=w15745)
        n9825 = call <vilib>:"MB Serial Master Query Write Multiple Registers (poly).vi"(0:w15747, 1:w15745, 2:w15741, 5:w15746, 6:w15748) -> (14:w15755, 19:w15754)  [unwired: 12 in, 1 out]
        n9826 = local write "TC2_open_loop_set"(i16? 0 ("TC2_open_loop_set")) -> ()
        n9827 = Build Array(i32? 49152 ("element")) -> (w15753)
        n9828 = call <vilib>:"MB Serial Master Query Write Multiple Registers (poly).vi"(0:w15755, 1:i16? 320 ("Starting Address"), 2:w15753, 5:w15754, 6:w15748) -> (14:w15759, 19:w15760)  [unwired: 12 in, 1 out]
        n9829 = Build Array(i32? 49407 ("element")) -> (w15756)
        n9830 = call <vilib>:"MB Serial Master Query Write Multiple Registers (poly).vi"(0:w15759, 1:i16? 320 ("Starting Address"), 2:w15756, 5:w15760, 6:w15748) -> (14:w15750, 19:w15749)  [unwired: 12 in, 1 out]
      }
      frame #3 {
        w15770 = data[3B] ("Serial Parameters")
        n9831 = Type Cast(type=data[3B], x="TC2_close_loop_coefficient") -> (*(type *) &x=w15762)
        n9832 = Build Array(w15762) -> (w15763)
        n9833 = Increment(x=i16? 84) -> (x+1=w15767)
        n9834 = local write "TC2_close_loop_set"(i16? 0 ("TC2_close_loop_set")) -> ()
        n9835 = call <vilib>:"MB Serial Master Query Write Multiple Registers (poly).vi"(0:w15769, 1:w15767, 2:w15763, 5:w15768, 6:w15770) -> (14:w15777, 19:w15776)  [unwired: 12 in, 1 out]
        n9836 = Build Array(i32? 49152 ("element")) -> (w15775)
        n9837 = call <vilib>:"MB Serial Master Query Write Multiple Registers (poly).vi"(0:w15777, 1:i16? 320 ("Starting Address"), 2:w15775, 5:w15776, 6:w15770) -> (14:w15781, 19:w15782)  [unwired: 12 in, 1 out]
        n9838 = Build Array(i32? 49407 ("element")) -> (w15778)
        n9839 = call <vilib>:"MB Serial Master Query Write Multiple Registers (poly).vi"(0:w15781, 1:i16? 320 ("Starting Address"), 2:w15778, 5:w15782, 6:w15770) -> (14:w15772, 19:w15771)  [unwired: 12 in, 1 out]
      }
      frame #4 {
        w15792 = data[3B] ("Serial Parameters")
        n9840 = Type Cast(type=data[3B], x="TC2_P_coefficient") -> (*(type *) &x=w15784)
        n9841 = Build Array(w15784) -> (w15785)
        n9842 = Increment(x=i16? 108) -> (x+1=w15789)
        n9843 = call <vilib>:"MB Serial Master Query Write Multiple Registers (poly).vi"(0:w15791, 1:w15789, 2:w15785, 5:w15790, 6:w15792) -> (14:w15799, 19:w15798)  [unwired: 12 in, 1 out]
        n9844 = local write "TC2_P_set"(i16? 0 ("TC2_P_set")) -> ()
        n9845 = Build Array(i32? 49152 ("element")) -> (w15797)
        n9846 = call <vilib>:"MB Serial Master Query Write Multiple Registers (poly).vi"(0:w15799, 1:i16? 320 ("Starting Address"), 2:w15797, 5:w15798, 6:w15792) -> (14:w15803, 19:w15804)  [unwired: 12 in, 1 out]
        n9847 = Build Array(i32? 49407 ("element")) -> (w15800)
        n9848 = call <vilib>:"MB Serial Master Query Write Multiple Registers (poly).vi"(0:w15803, 1:i16? 320 ("Starting Address"), 2:w15800, 5:w15804, 6:w15792) -> (14:w15794, 19:w15793)  [unwired: 12 in, 1 out]
      }
      frame #5 {
        w15814 = data[3B] ("Serial Parameters")
        n9849 = Type Cast(type=data[3B], x="TC2_I_coefficient") -> (*(type *) &x=w15806)
        n9850 = Build Array(w15806) -> (w15807)
        n9851 = Increment(x=i16? 110) -> (x+1=w15811)
        n9852 = call <vilib>:"MB Serial Master Query Write Multiple Registers (poly).vi"(0:w15813, 1:w15811, 2:w15807, 5:w15812, 6:w15814) -> (14:w15821, 19:w15820)  [unwired: 12 in, 1 out]
        n9853 = local write "TC2_I_set"(i16? 0 ("TC2_I_set")) -> ()
        n9854 = Build Array(i32? 49152 ("element")) -> (w15819)
        n9855 = call <vilib>:"MB Serial Master Query Write Multiple Registers (poly).vi"(0:w15821, 1:i16? 320 ("Starting Address"), 2:w15819, 5:w15820, 6:w15814) -> (14:w15825, 19:w15826)  [unwired: 12 in, 1 out]
        n9856 = Build Array(i32? 49407 ("element")) -> (w15822)
        n9857 = call <vilib>:"MB Serial Master Query Write Multiple Registers (poly).vi"(0:w15825, 1:i16? 320 ("Starting Address"), 2:w15822, 5:w15826, 6:w15814) -> (14:w15816, 19:w15815)  [unwired: 12 in, 1 out]
      }
      frame #6 {
        w15836 = data[3B] ("Serial Parameters")
        n9858 = Type Cast(type=data[3B], x="TC2_D_coefficient") -> (*(type *) &x=w15828)
        n9859 = Build Array(w15828) -> (w15829)
        n9860 = Increment(x=i16? 112) -> (x+1=w15833)
        n9861 = call <vilib>:"MB Serial Master Query Write Multiple Registers (poly).vi"(0:w15835, 1:w15833, 2:w15829, 5:w15834, 6:w15836) -> (14:w15843, 19:w15842)  [unwired: 12 in, 1 out]
        n9862 = local write "TC2_D_set"(i16? 0 ("TC2_D_set")) -> ()
        n9863 = Build Array(i32? 49152 ("element")) -> (w15841)
        n9864 = call <vilib>:"MB Serial Master Query Write Multiple Registers (poly).vi"(0:w15843, 1:i16? 320 ("Starting Address"), 2:w15841, 5:w15842, 6:w15836) -> (14:w15847, 19:w15848)  [unwired: 12 in, 1 out]
        n9865 = Build Array(i32? 49407 ("element")) -> (w15844)
        n9866 = call <vilib>:"MB Serial Master Query Write Multiple Registers (poly).vi"(0:w15847, 1:i16? 320 ("Starting Address"), 2:w15844, 5:w15848, 6:w15836) -> (14:w15838, 19:w15837)  [unwired: 12 in, 1 out]
      }
      frame #7 {
        w15858 = data[3B] ("Serial Parameters")
        n9867 = Type Cast(type=data[3B], x="TC2_speed_gain_value") -> (*(type *) &x=w15851)
        n9868 = Build Array(w15851) -> (w15852)
        n9869 = Increment(x=i16? 126) -> (x+1=w15856)
        n9870 = local write "TC2_speed_gain_set"(i16? 0 ("TC2_speed_gain_set")) -> ()
        n9871 = call <vilib>:"MB Serial Master Query Write Multiple Registers (poly).vi"(0:w15857, 1:w15856, 2:w15852, 5:w15850, 6:w15858) -> (14:w15865, 19:w15864)  [unwired: 12 in, 1 out]
        n9872 = Build Array(i32? 49152 ("element")) -> (w15863)
        n9873 = call <vilib>:"MB Serial Master Query Write Multiple Registers (poly).vi"(0:w15865, 1:i16? 320 ("Starting Address"), 2:w15863, 5:w15864, 6:w15858) -> (14:w15869, 19:w15870)  [unwired: 12 in, 1 out]
        n9874 = Build Array(i32? 49407 ("element")) -> (w15866)
        n9875 = call <vilib>:"MB Serial Master Query Write Multiple Registers (poly).vi"(0:w15869, 1:i16? 320 ("Starting Address"), 2:w15866, 5:w15870, 6:w15858) -> (14:w15860, 19:w15859)  [unwired: 12 in, 1 out]
      }
      frame #8 {
        w15880 = data[3B] ("Serial Parameters")
        n9876 = Type Cast(type=data[3B], x="TC2_speed_coefficient_value") -> (*(type *) &x=w15872)
        n9877 = Build Array(w15872) -> (w15873)
        n9878 = Increment(x=i16? 128) -> (x+1=w15877)
        n9879 = call <vilib>:"MB Serial Master Query Write Multiple Registers (poly).vi"(0:w15879, 1:w15877, 2:w15873, 5:w15878, 6:w15880) -> (14:w15887, 19:w15886)  [unwired: 12 in, 1 out]
        n9880 = local write "TC2_speed_coefficient_set"(i16? 0 ("TC2_speed_coefficient_set")) -> ()
        n9881 = Build Array(i32? 49152 ("element")) -> (w15885)
        n9882 = call <vilib>:"MB Serial Master Query Write Multiple Registers (poly).vi"(0:w15887, 1:i16? 320 ("Starting Address"), 2:w15885, 5:w15886, 6:w15880) -> (14:w15891, 19:w15892)  [unwired: 12 in, 1 out]